vi "HFRR ADV v038.vi"() -> ()   [LabVIEW 2025] (continued)
            n2155 = Bundle "Bundle"(w2346, w2342) -> (w2348:cluster{dbl[], dbl[]})  [unwired: 1 in]
            n2156 = Bundle "Bundle"(w2311, w2310) -> (w2318:cluster{dbl[], dbl[]})  [unwired: 1 in]
            n2157 = Bundle "Bundle"(w2344, w2340) -> (w2350:cluster{dbl[], dbl[]})  [unwired: 1 in]
            n2158 = Bundle "Bundle"(w2311, w2344) -> (w2454:cluster{dbl[], dbl[]})  [unwired: 1 in]
            n2159 = Bundle "Bundle"(w2311, w2340) -> (w2378:cluster{dbl[], dbl[]})  [unwired: 1 in]
            n2160 = Bundle "Bundle"(w2311, w2399) -> (w2464:cluster{dbl[], dbl[]})  [unwired: 1 in]
            n2161 = Bundle "Bundle"(w2311, w2394) -> (w2402:cluster{dbl[], dbl[]})  [unwired: 1 in]
            n2162 = Bundle "Bundle"(w2311, w2425) -> (w2449:cluster{dbl[], dbl[]})  [unwired: 1 in]
            n2163 = Bundle "Bundle"(w2345, w2341) -> (w2349:cluster{dbl[], dbl[]})  [unwired: 1 in]
            n2164 = Bundle "Bundle"(w2313, w2312) -> (w2319:cluster{dbl[], dbl[]})  [unwired: 1 in]
            n2165 = Bundle "Bundle"(w2313, w2345) -> (w2456:cluster{dbl[], dbl[]})  [unwired: 1 in]
            n2166 = Bundle "Bundle"(w2313, w2341) -> (w2379:cluster{dbl[], dbl[]})  [unwired: 1 in]
            n2167 = Bundle "Bundle"(w2313, w2395) -> (w2403:cluster{dbl[], dbl[]})  [unwired: 1 in]
            n2168 = Bundle "Bundle"(w2313, w2397) -> (w2465:cluster{dbl[], dbl[]})  [unwired: 1 in]
            n2169 = Bundle "Bundle"(w2313, w2434) -> (w2447:cluster{dbl[], dbl[]})  [unwired: 1 in]
            n2170 = Bundle "Bundle"(w2343, w2339) -> (w2351:cluster{dbl[], dbl[]})  [unwired: 1 in]
            n2171 = Bundle "Bundle"(w2309, w2308) -> (w2317:cluster{dbl[], dbl[]})  [unwired: 1 in]
            n2172 = Bundle "Bundle"(w2309, w2343) -> (w2455:cluster{dbl[], dbl[]})  [unwired: 1 in]
            n2173 = Bundle "Bundle"(w2309, w2339) -> (w2377:cluster{dbl[], dbl[]})  [unwired: 1 in]
            n2174 = Bundle "Bundle"(w2309, w2393) -> (w2401:cluster{dbl[], dbl[]})  [unwired: 1 in]
            n2175 = Bundle "Bundle"(w2309, w2398) -> (w2463:cluster{dbl[], dbl[]})  [unwired: 1 in]
            n2176 = Bundle "Bundle"(w2309, w2416) -> (w2448:cluster{dbl[], dbl[]})  [unwired: 1 in]
            n2177 = call-poly <vilib>:"Mean.vi"("X"=w2396) -> ("mean"=→"CP1":dbl)  [unwired: 1 out]
            n2178 = call-poly <vilib>:"Mean.vi"("X"=w2337) -> ("mean"=→"КОФ2 3":dbl)  [unwired: 1 out]
            n2179 = call-poly <vilib>:"Mean.vi"("X"=w2395) -> ("mean"=→"CP2":dbl)  [unwired: 1 out]
            n2180 = call-poly <vilib>:"Mean.vi"("X"=w2397) -> ("mean"=→"КОФ2":dbl)  [unwired: 1 out]
            n2181 = call-poly <vilib>:"Mean.vi"("X"=w2335) -> ("mean"=→"КОФ2 5":dbl)  [unwired: 1 out]
            n2182 = call-poly <vilib>:"Mean.vi"("X"=w2393) -> ("mean"=→"CP4":dbl)  [unwired: 1 out]
            n2183 = call-poly <vilib>:"Mean.vi"("X"=w2398) -> ("mean"=→"КОФ4":dbl)  [unwired: 1 out]
            n2184 = Bundle "Bundle"(w2315, w2342) -> (w2306:cluster{dbl[], dbl[]})  [unwired: 1 in]
            n2185 = Bundle "Bundle"(w2315, w2396) -> (w2329:cluster{dbl[], dbl[]})  [unwired: 1 in]
            n2186 = Build Array "Build Array"(w2306, w2329) -> (w2332:cluster{dbl[], dbl[]}[])
            "XY Graph 17" <- w2332
            n2187 = Build Array "Build Array"(w2320, w2319, w2318, w2317) -> (→"Frequency ( Hz )":cluster{dbl[], dbl[]}[])
            n2188 = Build Array "Build Array"(w2348, w2349, w2350, w2351) -> (→"Air Temp ( °C ) vs Humidity ( % RH )":cluster{dbl[], dbl[]}[])
            n2189 = Build Array "Build Array"(w2333, w2456, w2454, w2455) -> (→"Air Temperature  ( °C )":cluster{dbl[], dbl[]}[])
            n2190 = Build Array "Build Array"(w2306, w2379, w2378, w2377) -> (→"Humidity ( %RH )":cluster{dbl[], dbl[]}[])
            n2191 = Build Array "Build Array"(w2334, w2465, w2464, w2463) -> (→"Coefficient Of Friction":cluster{dbl[], dbl[]}[])
            n2192 = Build Array "Build Array"(w2329, w2403, w2402, w2401) -> (→"Sample Temperature ( °C )":cluster{dbl[], dbl[]}[])
            n2193 = Build Array "Build Array"(w2307, w2447, w2449, w2448) -> (→"XY Graph 13":cluster{dbl[], dbl[]}[])
            n2194 = Bundle "Bundle"(w2315, w2338) -> (w2360:cluster{dbl[], dbl[]})  [unwired: 1 in]
            n2195 = Bundle "Bundle"(w2311, w2336) -> (w2358:cluster{dbl[], dbl[]})  [unwired: 1 in]
            n2196 = Bundle "Bundle"(w2313, w2337) -> (w2359:cluster{dbl[], dbl[]})  [unwired: 1 in]
            n2197 = Bundle "Bundle"(w2309, w2335) -> (w2357:cluster{dbl[], dbl[]})  [unwired: 1 in]
            n2198 = Build Array "Build Array"(w2360, w2359, w2358, w2357) -> (→"Stroke ( mm )":cluster{dbl[], dbl[]}[])
            n2199 = local write "XY Graph 16"(w2332) -> ()
          }
          frame #2 {
          }
          frame #3 {
            n2200 = local write "Numeric 8"(0 ("Numeric 8")) -> ()
            n2201 = local write "Numeric 11"(0 ("Numeric 11")) -> ()
            n2202 = local write "Numeric 12"(0 ("Numeric 12")) -> ()
            n2203 = local write "Numeric 13"(0 ("Numeric 13")) -> ()
            n2204 = property on="OPEN" class="Bool (strict)"("Visible"=TRUE) -> ()  [unwired: 2 in, 2 out]
            n2205 = local read "String Control 2"() -> (w2632:string)
            n2206 = local read "String Control 4"() -> (w2631:string)
            n2207 = local read "String Control 6"() -> (w2630:string)
            n2208 = local read "String Control 8"() -> (w2629:string)
            n2209 = Match Pattern(string=w2632, regular expression="Samples / cycle :- ") -> (after substring=w2646:string)  [unwired: 1 in, 3 out]
            n2210 = Match Pattern(string=w2632, regular expression="Frequency :- ") -> (after substring=w2665:string)  [unwired: 1 in, 3 out]
            n2211 = Match Pattern(string=w2631, regular expression="Samples / cycle :- ") -> (after substring=w2642:string)  [unwired: 1 in, 3 out]
            n2212 = Match Pattern(string=w2631, regular expression="Frequency :- ") -> (after substring=w2660:string)  [unwired: 1 in, 3 out]
            n2213 = Match Pattern(string=w2630, regular expression="Samples / cycle :- ") -> (after substring=w2638:string)  [unwired: 1 in, 3 out]
            n2214 = Match Pattern(string=w2630, regular expression="Frequency :- ") -> (after substring=w2655:string)  [unwired: 1 in, 3 out]
            n2215 = Match Pattern(string=w2629, regular expression="Samples / cycle :- ") -> (after substring=w2634:string)  [unwired: 1 in, 3 out]
            n2216 = Match Pattern(string=w2629, regular expression="Frequency :- ") -> (after substring=w2650:string)  [unwired: 1 in, 3 out]
            n2217 = String Subset(string=w2646, length (rest)=6 ("length (rest)")) -> (substring=w2648:string)  [unwired: 1 in]
            n2218 = String Subset(string=w2665, length (rest)=9 ("length (rest)")) -> (substring=w2667:string)  [unwired: 1 in]
            n2219 = String Subset(string=w2642, length (rest)=6 ("length (rest)")) -> (substring=w2644:string)  [unwired: 1 in]
            n2220 = String Subset(string=w2660, length (rest)=9 ("length (rest)")) -> (substring=w2662:string)  [unwired: 1 in]
            n2221 = String Subset(string=w2638, length (rest)=6 ("length (rest)")) -> (substring=w2640:string)  [unwired: 1 in]
            n2222 = String Subset(string=w2655, length (rest)=9 ("length (rest)")) -> (substring=w2657:string)  [unwired: 1 in]
            n2223 = String Subset(string=w2634, length (rest)=6 ("length (rest)")) -> (substring=w2636:string)  [unwired: 1 in]
            n2224 = String Subset(string=w2650, length (rest)=9 ("length (rest)")) -> (substring=w2652:string)  [unwired: 1 in]
            n2225 = Fract/Exp String To Number(string=w2648) -> (number=w2628:dbl)  [unwired: 3 in, 1 out]
            n2226 = Fract/Exp String To Number(string=w2667) -> (number=w2668:dbl)  [unwired: 3 in, 1 out]
            n2227 = Fract/Exp String To Number(string=w2644) -> (number=w2627:dbl)  [unwired: 3 in, 1 out]
            n2228 = Fract/Exp String To Number(string=w2662) -> (number=w2663:dbl)  [unwired: 3 in, 1 out]
            n2229 = Fract/Exp String To Number(string=w2640) -> (number=w2626:dbl)  [unwired: 3 in, 1 out]
            n2230 = Fract/Exp String To Number(string=w2657) -> (number=w2658:dbl)  [unwired: 3 in, 1 out]
            n2231 = Fract/Exp String To Number(string=w2636) -> (number=w2625:dbl)  [unwired: 3 in, 1 out]
            n2232 = Fract/Exp String To Number(string=w2652) -> (number=w2653:dbl)  [unwired: 3 in, 1 out]
            n2233 = local write "sample1"(w2628) -> ()
            n2234 = local write "freq1"(w2668) -> ()
            n2235 = local write "sample2"(w2627) -> ()
            n2236 = local write "freq2"(w2663) -> ()
            n2237 = local write "sample3"(w2626) -> ()
            n2238 = local write "freq3"(w2658) -> ()
            n2239 = local write "sample4"(w2625) -> ()
            n2240 = local write "freq 4"(w2653) -> ()
          }
        }
      }
    }
    n2241 = case shown="True" w2226 {
      selector: w2226 -> [_ w2245]
      frame False {
      }
      frame True {
        n2242 = Not(x=w2245) -> (.not. x?=w2241:bool)
        n2243 = local write "service 3"(w2241) -> ()
        n2244 = local write "OPEN 6"(w2241) -> ()
        n2245 = call <vilib>:"System Exec.vi"("wait until completion? (T)"=TRUE, "command line"="C:\\LAB-IQ\\Scar View.exe") -> ("error out"=→"error out 5":errorcluster)  [unwired: 6 in, 3 out]
      }
    }
    n2246 = case shown="\"Acquire\", Default" w2235 {
      frame "Acquire", Default {
        # "Elapsed time\ncof\nstroke\nAir temp\nTemp\nHumidity"
        n2247 = disable-structure shown="Disabled" {
          frame Disabled {
            n2248 = local read "Flag"() -> (w2944:dbl)
            n2249 = local read "RUN"() -> (w2941:bool)
            n2250 = Not(x=w2941) -> (.not. x?=w2940:bool)
            n2251 = Equal?(x=w2944, y=10.0) -> (x = y?=w2942:bool)
            n2252 = And(x=w2942, y=w2940) -> (x .and. y?=w2939:bool)
            n2253 = case shown="True" w2939 {
              frame False {
              }
              frame True {
                w2945 = FALSE ("Heater Button")
                n2254 = local write "Humidity"(w2945) -> ()
                n2255 = local write "Heater Button"(w2945) -> ()
              }
            }
          }
          frame Enabled {
          }
        }
        n2256 = disable-structure shown="Disabled" {
          frame Disabled {
            n2257 = case shown="True" {
              selector: _ -> [_ _]
              frame False {
              }
              frame True {
                w2990 = TRUE ("Heater")
                n2258 = local write "Humidity"(w2990) -> ()
                n2259 = local write "Heater Button"(w2990) -> ()
                n2260 = local read "TEST STANDARD"() -> (w2993:T3)
                n2261 = local read "TEST STANDARD"() -> (w2988:T3)
                n2262 = Equal?(x=w2993, y=enum16{"ASTM D6079", "ISO 12156", "Custom"}."ISO 12156" ("Test Standard")) -> (x = y?=w2991:bool)
                n2263 = Equal?(x=w2988, y=enum16{"ASTM D6079", "ISO 12156", "Custom"}."ASTM D6079" ("Test Standard")) -> (x = y?=w2987:bool)
                n2264 = case shown="True" w2991 {
                  frame False {
                  }
                  frame True {
                    n2265 = local write "airtempflg"(FALSE ("airtempflg")) -> ()
                    n2266 = local write item#-1(TRUE ("Heater")) -> ()
                  }
                }
                n2267 = case shown="True" w2987 {
                  frame False {
                  }
                  frame True {
                    n2268 = local write "airtempflg"(TRUE ("airtempflg")) -> ()
                    n2269 = local write item#-1(FALSE ("Heater")) -> ()
                  }
                }
              }
            }
          }
          frame Enabled {
          }
        }
        n2270 = stacked-sequence {
          frame #0 {
            n2271 = case shown="True" "RST FF" {
              frame False {
              }
              frame True {
                w3007 = 0.0 ("X Scale.Range:Maximum")
                n2272 = property on="Frictional Force ( N )" class="WFChart (strict)"("XScale.Maximum"=600.0 ("X Scale.Range:Maximum"), "XScale.Minimum"=w3007, "YScale.Maximum"=10.0 ("Y Scale.Range:Maximum"), "YScale.Minimum"=w3007) -> ()  [unwired: 2 in, 2 out]
              }
            }
          }
          frame #1 {
            n2273 = case shown="True" "RST TEMP" {
              frame False {
              }
              frame True {
                n2274 = property on="Temperature ( Deg C )" class="WFChart (strict)"("XScale.Minimum"=0.0 ("X Scale.Range:Minimum"), "XScale.Maximum"=600.0 ("X Scale.Range:Maximum"), "YScale.Minimum"=0.0 ("Y Scale.Range:Minimum"), "YScale.Maximum"=100.0 ("Y Scale.Range:Maximum")) -> ()  [unwired: 2 in, 2 out]
              }
            }
          }
          frame #2 {
            n2275 = case shown="True" "RSTCOF" {
              frame False {
              }
              frame True {
                n2276 = property on="Coefficient of Friction" class="WFChart (strict)"("XScale.Minimum"=0.0 ("X Scale.Range:Minimum"), "XScale.Maximum"=600.0 ("X Scale.Range:Maximum"), "YScale.Maximum"=1.0 ("X Scale.Range:Minimum"), "YScale.Minimum"=0.0 ("X Scale.Range:Minimum")) -> ()  [unwired: 2 in, 2 out]
              }
            }
          }
          frame #3 {
            n2277 = case shown="True" "RSTCOF 2" {
              frame False {
              }
              frame True {
                (unwired) 100.0 ("Y Scale.Range:Maximum")
                (unwired) 0.0 ("Y Scale.Range:Minimum")
                (unwired) 600.0 ("X Scale.Range:Maximum")
                (unwired) 0.0 ("X Scale.Range:Minimum")
              }
            }
          }
          frame #4 {
            n2278 = case shown="True" "RSTCOF 3" {
              frame False {
              }
              frame True {
                n2279 = property on="Electrical Contact Resistance ( % )" class="WFChart (strict)"("XScale.Minimum"=0.0 ("X Scale.Range:Minimum"), "XScale.Maximum"=600.0 ("X Scale.Range:Maximum"), "YScale.Minimum"=0.0 ("Y Scale.Range:Minimum"), "YScale.Maximum"=100.0 ("Y Scale.Range:Maximum")) -> ()  [unwired: 2 in, 2 out]
              }
            }
          }
        }
        n2280 = local read "RUN"() -> (w2934:bool)
        n2281 = case shown="False" w2934 {
          frame False {
          }
          frame True {
          }
        }
        n2282 = local read "RUN"() -> (w2938:bool)
        n2283 = case shown="False" w2938 {
          tunnel: [FALSE ("TEST RUNNING") TRUE ("TEST RUNNING")] -> w2937
          frame False {
            w3026 = 0.0 ("Flag")
            n2284 = local write "Elapsed time"(0.0 ("elapsedtime")) -> ()
            n2285 = local write "Time Remaining"(w3026) -> ()
            n2286 = local write "Flag"(w3026) -> ()
            n2287 = local write "Remaining Time"(w3026) -> ()
          }
          frame True {
            n2288 = local write "Flag"(10.0 ("Flag")) -> ()
          }
        }
        n2289 = local read "AIR TEMP"() -> (w2932:dbl)
        n2290 = Greater Or Equal?(x=w2932, y=15.0) -> (x >= y?=w2933:bool)
        "powstat" <- w2933
        n2291 = case shown="True" "Save & Continue" {
          frame False {
          }
          frame True {
            n2292 = local read "USER ID"() -> (w3330:string)
            n2293 = local read "FILE"() -> (w3338:string)
            n2294 = String Length(string=w3338) -> (length=w3336:i32)
            n2295 = String Length(string=w3330) -> (length=w3333:i32)
            n2296 = Greater?(x=w3336, y=0) -> (0:w3335:bool)
            n2297 = Greater?(x=w3333, y=0) -> (0:w3332:bool)
            n2298 = And(x=w3335, y=w3332) -> (x .and. y?=w3331:bool)
            n2299 = case shown="True" w3331 {
              frame False {
                n2300 = stacked-sequence {
                  frame #0 {
                    n2301 = One Button Dialog(message="Please Enter a File Name and Operator ID to save data !", button name ("OK")="Ok") -> ()  [unwired: 1 out]
                  }
                  frame #1 {
                    n2302 = local write "Save & Continue"(FALSE ("OK Button")) -> ()
                  }
                }
                n2303 = local write "Save & Continue"(FALSE ("OK Button")) -> ()
              }
              frame True {
                n2304 = stacked-sequence {
                  frame #0 {
                    n2305 = local read "FILE"() -> (w3344:string)
                    n2306 = call "file check.vi"("file name in"=w3344) -> ("file name out"=w3343:string)  [unwired: 9 in, 1 out]
                    n2307 = call <vilib>:"Application Directory.vi"() -> ("Application Directory"=w3354:path)
                    n2308 = Build Path(base path=w3354, name or relative path="data") -> (appended path=w3353:path)
                    n2309 = call <vilib>:"Trim Whitespace.vi"("string"=w3343) -> ("trimmed string"=w3351:string)  [unwired: 1 in]
                    n2310 = call <vilib>:"Trim Whitespace.vi"("string"=w3343) -> ("trimmed string"=w3352:string)  [unwired: 1 in]
                    n2311 = List Folder(path=w3353) -> (folder names=w3349:string[])  [unwired: 3 in, 3 out]
                    n2312 = Match Pattern(string=w3351, regular expression="_(") -> (before substring=w3348:string)  [unwired: 1 in, 3 out]
                    n2313 = for {
                      tunnel: w3349 -> [w3363] mode=indexing
                      tunnel: w3348 -> [w3361]
                      shift-right: [w3359] -> w3346
                      shift-left: bool[] [] -> [w3360]
                      n2314 = Match Pattern(string=w3363, regular expression="_(") -> (before substring=w3362:string)  [unwired: 1 in, 3 out]
                      n2315 = Equal?(x=w3362, y=w3361) -> (x = y?=w3358:bool)
                      n2316 = case shown="True" w3358 {
                        tunnel: w3358 -> [_ w3366]
                        tunnel: w3360 -> [w3365 w3368]
                        tunnel: [w3365 w3367] -> w3359
                        frame False {
                        }
                        frame True {
                          n2317 = Insert Into Array(array=w3368, new element=w3366) -> (w3367:bool[])  [unwired: 1 in]
                        }
                      }
                    }
                    n2318 = Equal?(x=w3349, y=w3348) -> (x = y?=w3357:bool[])
                    n2319 = Or Array Elements(Boolean array=w3357) -> (logical OR=w3356:bool)
                    n2320 = Array Size(array=w3346) -> (size(s)=w3345:i32)
                    n2321 = case shown="True" w3356 {
                      tunnel: w3352 -> [_ w3376]
                      tunnel: w3345 -> [_ w3369]
                      frame False {
                      }
                      frame True {
                        n2322 = Number To Decimal String(number=w3369) -> (decimal integer string=w3372:string)  [unwired: 1 in]
                        n2323 = Search/Split String(string=w3376, search string/char (-)="_(" ("regular expression")) -> (substring before match=w3374:string)  [unwired: 1 in, 2 out]
                        n2324 = Concatenate Strings(w3374, "_(" ("regular expression"), w3372, ")" ("regular expression")) -> (w3370:string)
                        n2325 = local write "FILE"(w3370) -> ()
                      }
                    }
                  }
                  frame #1 {
                    w3379 = 0.0
                    w3392 = cluster{"y":dbl, dbl, "y":dbl}[] [] ("History Data")
                    w3393 = FALSE ("Heater Button")
                    (unwired) ")!" ("string")
                    (unwired) ")" ("string")
                    w3391 = dbl[] [] ("History Data")
                    w3397 = "\r"
                    # "C:\\WinDucom\\Data\\"
                    # "C:\\LAB-IQ-NXT\\data"
                    n2326 = local write "Humidity ( %RH )"(w3379) -> ()
                    n2327 = local write "Frequency ( Hz )"(w3379) -> ()
                    n2328 = local write "Stroke 3"(w3379) -> ()
                    n2329 = local write "speedop"(0.0 ("PIDclk 2")) -> ()
                    n2330 = local write "Set Temp 2"(65.0 ("Set Temp 2")) -> ()
                    n2331 = local write "AIR TEMP"(w3379) -> ()
                    n2332 = local write "clk"(0.0 ("clk")) -> ()
                    n2333 = local write "Stroke 4"(w3379) -> ()
                    n2334 = local write "COF 2"(w3379) -> ()
                    n2335 = local write "TEMP"(w3379) -> ()
                    n2336 = local write "ecr 3"(w3379) -> ()
                    n2337 = local write "FF 3"(w3379) -> ()
                    n2338 = local write "FF 2"(w3379) -> ()
                    n2339 = property on="Coefficient of Friction" class="WFChart (strict)"("History Data"=w3391) -> ()  [unwired: 2 in, 2 out]
                    n2340 = property on="Coefficient of Friction" class="WFChart (strict)"("History Data"=w3391) -> ()  [unwired: 2 in, 2 out]
                    n2341 = property on="Frictional Force ( N )" class="WFChart (strict)"("History Data"=w3391) -> ()  [unwired: 2 in, 2 out]
                    n2342 = property on="Electrical Contact Resistance ( % )" class="WFChart (strict)"("History Data"=w3391) -> ()  [unwired: 2 in, 2 out]
                    n2343 = property on="Electrical Contact Resistance ( % )" class="WFChart (strict)"("History Data"=w3391) -> ()  [unwired: 2 in, 2 out]
                    n2344 = property on="Temperature ( Deg C )" class="WFChart (strict)"("History Data"=w3391) -> ()  [unwired: 2 in, 2 out]
                    n2345 = property on="Frictional Force ( N )" class="WFChart (strict)"("History Data"=w3391) -> ()  [unwired: 2 in, 2 out]
                    n2346 = property on="Coefficient of Friction" class="WFChart (strict)"("History Data"=w3391) -> ()  [unwired: 2 in, 2 out]
                    n2347 = property on="Frictional Force ( N )" class="WFChart (strict)"("History Data"=w3391) -> ()  [unwired: 2 in, 2 out]
                    n2348 = property on="Electrical Contact Resistance ( % )" class="WFChart (strict)"("History Data"=w3391) -> ()  [unwired: 2 in, 2 out]
                    n2349 = property on="Temperature ( Deg C )" class="WFChart (strict)"("History Data"=w3391) -> ()  [unwired: 2 in, 2 out]
                    n2350 = property on="Stroke ( mm )" class="WFChart (strict)"("History Data"=w3392) -> ()  [unwired: 2 in, 2 out]
                    n2351 = property on="Stroke ( mm )" class="WFChart (strict)"("History Data"=w3392) -> ()  [unwired: 2 in, 2 out]
                    n2352 = local write "Humidity"(w3393) -> ()
                    n2353 = local write "Heater Button"(w3393) -> ()
                    n2354 = local read "FILE"() -> (w3387:string)
                    n2355 = disable-structure shown="Enabled" {
                      disable-tunnel: [w3431 _] -> w3378
                      frame Enabled {
                        n2356 = local read "NORMAL LOAD"() -> (w3431:dbl)
                      }
                      frame Disabled {
                      }
                    }
                    n2357 = call "file check.vi"("file name in"=w3387) -> ("error out"=w3390:errorcluster, "file name out"=w3384:string)  [unwired: 9 in]
                    n2358 = call "FILE PATH CREATION.vi"("error in"=w3390, "FILE NAME :"=w3384) -> ("FILE OUT"=w3383:path)  [unwired: 8 in, 1 out]
                    n2359 = Concatenate Strings(w3384, ".dgf" ("Substring")) -> (w3389:string)
                    n2360 = Concatenate Strings(w3384, ".duf" ("Substring")) -> (w3385:string)
                    n2361 = Multiply(x=w3378, y=1.0) -> (x*y=w3410:dbl)
                    n2362 = Build Path(base path=w3383, name or relative path=w3389) -> (appended path=w3382:path)
                    n2363 = Build Path(base path=w3383, name or relative path=w3385) -> (appended path=w3381:path)
                    n2364 = Number To Fractional String(number=w3410, width (-)=i16 5, precision (6)=i16 2) -> (F-format string=w3418:string)  [unwired: 1 in]
                    n2365 = local read "tested by"() -> (w3377:string)
                    n2366 = local read "Fuel Discription :"() -> (w3406:string)
                    n2367 = local read "Batch Ref Num :"() -> (w3395:string)
                    n2368 = Get Date/Time String(date format (0)=enum16{"short", "long", "abbreviated"}."short") -> (date string=w3429:string, time string=w3426:string)  [unwired: 2 in]
                    n2369 = local read "Remarks :"() -> (w3405:string)
                    n2370 = Concatenate Strings("Load :- " ("Substring"), w3418, " grams ," ("Substring")) -> (w3417:string)
                    n2371 = local read "String 41"() -> (w3398:string)
                    n2372 = Concatenate Strings(w3406) -> (w3407:string)
                    n2373 = Concatenate Strings(w3395) -> (w3394:string)
                    n2374 = Concatenate Strings(w3377) -> (w3401:string)
                    n2375 = Concatenate Strings("(" ("Substring"), w3429, ")" ("Substring"), w3426) -> (w3400:string)
                    "concatenated string" <- w3400
                    n2376 = Concatenate Strings(w3405, "," ("string")) -> (w3404:string)
                    n2377 = Concatenate Strings("  TIME;      COF;       STROKE;     AIR TEMP;  TEMP;  HUMIDITY;  ECR; PID-OUT; FREQUENCY" ("Substring"), "\r") -> (w3413:string)
                    n2378 = Concatenate Strings(w3398, w3397, "Fuel Discription :-" ("Substring"), w3407, w3397, w3417, w3397, "Batch Ref Num :-" ("Substring"), w3394, w3397, " Remarks :- " ("Substring"), w3404, w3397, " Date :- " ("Substring"), w3400, w3397, "Tested By :-" ("Substring"), w3401) -> (w3411:string)
                    "REMARKS" <- w3411
                    n2379 = call <vilib>:"Write Characters To File.vi"("append to file? (new file:F)"=FALSE, "character string"=w3413, "file path (dialog if empty)"=w3382) -> ()  [unwired: 2 in, 1 out]
                    n2380 = call <vilib>:"Write Characters To File.vi"("append to file? (new file:F)"=FALSE, "character string"=w3411, "file path (dialog if empty)"=w3381) -> ()  [unwired: 2 in, 1 out]
                  }
                  frame #2 {
                    n2381 = local write "Cycles elapsed"(0 ("Cycles elapsed")) -> ()
                    n2382 = local write "cyclecount"(0 ("cyclecount")) -> ()
                    n2383 = local write "Save & Continue"(FALSE ("OK")) -> ()
                    n2384 = local write "autostrtflg"(TRUE ("autostrtflg")) -> ()
                    n2385 = local write "Save"(FALSE ("Save")) -> ()
                    n2386 = Get Date/Time In Seconds() -> (seconds since 1Jan1904=w3436:timestamp)
                    n2387 = To Double Precision Float(number=w3436) -> (double precision float=w3435:dbl)
                    n2388 = local write "acq timer"(w3435) -> ()
                    n2389 = One Button Dialog(message="Please ensure sample is mounted properly and machine is ready in all aspects for testing !", button name ("OK")="Ok") -> ()  [unwired: 1 out]
                  }
                  frame #3 {
                    n2390 = stacked-sequence {
                      frame #0 {
                        n2391 = local write "Main Dashboard Buttons"(T1."Dashboard" ("Main Dashboard Buttons")) -> ()
                        n2392 = local write "Main Tab"(T2."Acquire" ("Main Tab")) -> ()
                      }
                      frame #1 {
                        n2393 = local write "EVENT LOG"("" ("EVENT LOG")) -> ()
                      }
                      frame #2 {
                        n2394 = Wait (ms)(milliseconds to wait=u32 50) -> ()  [unwired: 1 out]
                      }
                      frame #3 {
                        n2395 = disable-structure shown="Disabled" {
                          frame Disabled {
                            n2396 = local read "EVENT LOG"() -> (w3448:string)
                            n2397 = call "Event Log.vi"("Content"="Test Details", "EVENT LOG"=w3448) -> ("EVENT LOG"=w3447:string)  [unwired: 8 in, 1 out]
                            n2398 = local write "EVENT LOG"(w3447) -> ()
                          }
                          frame Enabled {
                          }
                        }
                      }
                      frame #4 {
                        n2399 = Wait (ms)(milliseconds to wait=u32 50) -> ()  [unwired: 1 out]
                      }
                      frame #5 {
                        n2400 = local read "FILE"() -> (w3450:string)
                        n2401 = Concatenate Strings("File Name :" ("Content"), w3450) -> (w3451:string)
                        n2402 = local read "EVENT LOG"() -> (w3454:string)
                        n2403 = call "Event Log.vi"("Content"=w3451, "EVENT LOG"=w3454) -> ("EVENT LOG"=w3453:string)  [unwired: 8 in, 1 out]
                        n2404 = local write "EVENT LOG"(w3453) -> ()
                      }
                      frame #6 {
                        n2405 = Wait (ms)(milliseconds to wait=u32 50) -> ()  [unwired: 1 out]
                      }
                      frame #7 {
                        n2406 = local read "Batch Ref Num :"() -> (w3456:string)
                        n2407 = Concatenate Strings("Batch Ref No :" ("Content"), w3456) -> (w3457:string)
                        n2408 = local read "EVENT LOG"() -> (w3460:string)
                        n2409 = call "Event Log.vi"("Content"=w3457, "EVENT LOG"=w3460) -> ("EVENT LOG"=w3459:string)  [unwired: 8 in, 1 out]
                        n2410 = local write "EVENT LOG"(w3459) -> ()
                      }
                      frame #8 {
                        n2411 = Wait (ms)(milliseconds to wait=u32 50) -> ()  [unwired: 1 out]
                      }
                      frame #9 {
                        n2412 = local read "tested by"() -> (w3462:string)
                        n2413 = Concatenate Strings("Tested By :" ("Content"), w3462) -> (w3463:string)
                        n2414 = local read "EVENT LOG"() -> (w3466:string)
                        n2415 = call "Event Log.vi"("Content"=w3463, "EVENT LOG"=w3466) -> ("EVENT LOG"=w3465:string)  [unwired: 8 in, 1 out]
                        n2416 = local write "EVENT LOG"(w3465) -> ()
                      }
                      frame #10 {
                        n2417 = Wait (ms)(milliseconds to wait=u32 50) -> ()  [unwired: 1 out]
                      }
                      frame #11 {
                        n2418 = local read "TEST STANDARD"() -> (w3469:T3)
                        n2419 = case shown="\"ASTM D6079\", Default" w3469 {
                          tunnel: ["ASTM D6079" "ISO 12156" "CEC F-096-A-06" "Custom"] -> w3468
                          frame "ASTM D6079", Default {
                          }
                          frame "ISO 12156" {
                          }
                          frame "CEC F-096-A-06" {
                          }
                          frame "Custom" {
                          }
                        }
                        n2420 = Concatenate Strings("Test Standard :" ("Content"), w3468) -> (w3470:string)
                        n2421 = local read "EVENT LOG"() -> (w3473:string)
                        n2422 = call "Event Log.vi"("Content"=w3470, "EVENT LOG"=w3473) -> ("EVENT LOG"=w3472:string)  [unwired: 8 in, 1 out]
                        n2423 = local write "EVENT LOG"(w3472) -> ()
                      }
                      frame #12 {
                        n2424 = Wait (ms)(milliseconds to wait=u32 50) -> ()  [unwired: 1 out]
                      }
                      frame #13 {
                        n2425 = local read "Fuel Discription :"() -> (w3479:string)
                        n2426 = Concatenate Strings("Fuel Description :" ("Content"), w3479) -> (w3480:string)
                        n2427 = local read "EVENT LOG"() -> (w3483:string)
                        n2428 = call "Event Log.vi"("Content"=w3480, "EVENT LOG"=w3483) -> ("EVENT LOG"=w3482:string)  [unwired: 8 in, 1 out]
                        n2429 = local write "EVENT LOG"(w3482) -> ()
                      }
                      frame #14 {
                        n2430 = Wait (ms)(milliseconds to wait=u32 50) -> ()  [unwired: 1 out]
                      }
                      frame #15 {
                        n2431 = local read "Remarks :"() -> (w3485:string)
                        n2432 = Concatenate Strings("Remarks :" ("Content"), w3485) -> (w3486:string)
                        n2433 = local read "EVENT LOG"() -> (w3489:string)
                        n2434 = call "Event Log.vi"("Content"=w3486, "EVENT LOG"=w3489) -> ("EVENT LOG"=w3488:string)  [unwired: 8 in, 1 out]
                        n2435 = local write "EVENT LOG"(w3488) -> ()
                      }
                      frame #16 {
                        n2436 = Wait (ms)(milliseconds to wait=u32 50) -> ()  [unwired: 1 out]
                      }
                      frame #17 {
                        n2437 = local read "USER ID"() -> (w3491:string)
                        n2438 = Concatenate Strings("Operator ID :" ("Content"), w3491) -> (w3493:string)
                        n2439 = local read "EVENT LOG"() -> (w3495:string)
                        n2440 = call "Event Log.vi"("Content"=w3493, "EVENT LOG"=w3495) -> ("EVENT LOG"=w3494:string)  [unwired: 8 in, 1 out]
                        n2441 = local write "EVENT LOG"(w3494) -> ()
                      }
                      frame #18 {
                        n2442 = Wait (ms)(milliseconds to wait=u32 50) -> ()  [unwired: 1 out]
                      }
                      frame #19 {
                        n2443 = disable-structure shown="Disabled" {
                          frame Disabled {
                            n2444 = local read "EVENT LOG"() -> (w3499:string)
                            n2445 = call "Event Log.vi"("Content"="Test Parameter", "EVENT LOG"=w3499) -> ("EVENT LOG"=w3498:string)  [unwired: 8 in, 1 out]
                            n2446 = local write "EVENT LOG"(w3498) -> ()
                          }
                          frame Enabled {
                          }
                        }
                      }
                      frame #20 {
                        n2447 = Wait (ms)(milliseconds to wait=u32 50) -> ()  [unwired: 1 out]
                      }
                      frame #21 {
                        n2448 = local read "Set Hz"() -> (w3503:dbl)
                        n2449 = Number To Fractional String(number=w3503, precision (6)=i16 2) -> (F-format string=w3502:string)  [unwired: 2 in]
                        n2450 = Concatenate Strings("Set Frequency [Hz] :" ("Content"), w3502) -> (w3505:string)
                        n2451 = local read "EVENT LOG"() -> (w3507:string)
                        n2452 = call "Event Log.vi"("Content"=w3505, "EVENT LOG"=w3507) -> ("EVENT LOG"=w3506:string)  [unwired: 8 in, 1 out]
                        n2453 = local write "EVENT LOG"(w3506) -> ()
                      }
                      frame #22 {
                        n2454 = Wait (ms)(milliseconds to wait=u32 50) -> ()  [unwired: 1 out]
                      }
                      frame #23 {
                        n2455 = local read "NORMAL LOAD"() -> (w3510:dbl)
                        n2456 = Number To Fractional String(number=w3510, precision (6)=i16 2) -> (F-format string=w3511:string)  [unwired: 2 in]
                        n2457 = Concatenate Strings("Applied Load [grams] :" ("Content"), w3511) -> (w3513:string)
                        n2458 = local read "EVENT LOG"() -> (w3515:string)
                        n2459 = call "Event Log.vi"("Content"=w3513, "EVENT LOG"=w3515) -> ("EVENT LOG"=w3514:string)  [unwired: 8 in, 1 out]
                        n2460 = local write "EVENT LOG"(w3514) -> ()
                      }
                      frame #24 {
                        n2461 = Wait (ms)(milliseconds to wait=u32 50) -> ()  [unwired: 1 out]
                      }
                      frame #25 {
                        n2462 = local read "Set Strk"() -> (w3518:dbl)
                        n2463 = Number To Fractional String(number=w3518, precision (6)=i16 2) -> (F-format string=w3519:string)  [unwired: 2 in]
                        n2464 = Concatenate Strings("Set Stroke [mm] :" ("Content"), w3519) -> (w3521:string)
                        n2465 = local read "EVENT LOG"() -> (w3523:string)
                        n2466 = call "Event Log.vi"("Content"=w3521, "EVENT LOG"=w3523) -> ("EVENT LOG"=w3522:string)  [unwired: 8 in, 1 out]
                        n2467 = local write "EVENT LOG"(w3522) -> ()
                      }
                      frame #26 {
                        n2468 = Wait (ms)(milliseconds to wait=u32 50) -> ()  [unwired: 1 out]
                      }
                      frame #27 {
                        n2469 = local read "Set Temp"() -> (w3526:dbl)
                        n2470 = Number To Fractional String(number=w3526, precision (6)=i16 2) -> (F-format string=w3527:string)  [unwired: 2 in]
                        n2471 = Concatenate Strings("Set Temperature [deg C] :" ("Content"), w3527) -> (w3529:string)
                        n2472 = local read "EVENT LOG"() -> (w3531:string)
                        n2473 = call "Event Log.vi"("Content"=w3529, "EVENT LOG"=w3531) -> ("EVENT LOG"=w3530:string)  [unwired: 8 in, 1 out]
                        n2474 = local write "EVENT LOG"(w3530) -> ()
                      }
                      frame #28 {
                        n2475 = Wait (ms)(milliseconds to wait=u32 50) -> ()  [unwired: 1 out]
                      }
                      frame #29 {
                        n2476 = local read "Set Rh"() -> (w3534:dbl)
                        n2477 = Number To Fractional String(number=w3534, precision (6)=i16 2) -> (F-format string=w3535:string)  [unwired: 2 in]
                        n2478 = Concatenate Strings("Set Humidity [%RH] :" ("Content"), w3535) -> (w3537:string)
                        n2479 = local read "EVENT LOG"() -> (w3539:string)
                        n2480 = call "Event Log.vi"("Content"=w3537, "EVENT LOG"=w3539) -> ("EVENT LOG"=w3538:string)  [unwired: 8 in, 1 out]
                        n2481 = local write "EVENT LOG"(w3538) -> ()
                      }
                      frame #30 {
                        n2482 = Wait (ms)(milliseconds to wait=u32 50) -> ()  [unwired: 1 out]
                      }
                      frame #31 {
                        n2483 = local read "test time"() -> (w3542:dbl)
                        n2484 = Number To Fractional String(number=w3542, precision (6)=i16 1) -> (F-format string=w3543:string)  [unwired: 2 in]
                        n2485 = Concatenate Strings("Test Duration [mins] :" ("Content"), w3543) -> (w3545:string)
                        n2486 = local read "EVENT LOG"() -> (w3547:string)
                        n2487 = call "Event Log.vi"("Content"=w3545, "EVENT LOG"=w3547) -> ("EVENT LOG"=w3546:string)  [unwired: 8 in, 1 out]
                        n2488 = local write "EVENT LOG"(w3546) -> ()
                      }
                      frame #32 {
                        w3548 = dbl[] [] ("History Data")
                        w3549 = cluster{"y":dbl, dbl, "y":dbl}[] [] ("History Data")
                        w3550 = FALSE ("Visible")
                        n2489 = property on="Stroke ( mm )" class="WFChart (strict)"("History Data"=w3549) -> ()  [unwired: 2 in, 2 out]
                        n2490 = property on="Temperature ( Deg C )" class="WFChart (strict)"("History Data"=w3548) -> ()  [unwired: 2 in, 2 out]
                        n2491 = property on="Electrical Contact Resistance ( % )" class="WFChart (strict)"("History Data"=w3548) -> ()  [unwired: 2 in, 2 out]
                        n2492 = property on="Coefficient of Friction" class="WFChart (strict)"("History Data"=w3548) -> ()  [unwired: 2 in, 2 out]
                        n2493 = property on="Frictional Force ( N )" class="WFChart (strict)"("History Data"=w3548) -> ()  [unwired: 2 in, 2 out]
                        n2494 = property on="Coefficient of Friction" class="WFChart (strict)"("History Data"=w3548) -> ()  [unwired: 2 in, 2 out]
                        n2495 = property on="Frictional Force ( N )" class="WFChart (strict)"("History Data"=w3548) -> ()  [unwired: 2 in, 2 out]
                        n2496 = property on="Electrical Contact Resistance ( % )" class="WFChart (strict)"("History Data"=w3548) -> ()  [unwired: 2 in, 2 out]
                        n2497 = property on="Stroke ( mm )" class="WFChart (strict)"("History Data"=w3549) -> ()  [unwired: 2 in, 2 out]
                        n2498 = property on="Temperature ( Deg C )" class="WFChart (strict)"("History Data"=w3548) -> ()  [unwired: 2 in, 2 out]
                        n2499 = property on="Service Password Log" class="Str"("Visible"=w3550) -> ()  [unwired: 2 in, 2 out]
                        n2500 = property on="Password 3" class="Clust (strict)"("Visible"=w3550) -> ()  [unwired: 2 in, 2 out]
                      }
                    }
                    "TEST FILE NAM,E SAVED" <- TRUE ("TEST FILE NAM,E SAVED")
                  }
                }
              }
            }
          }
        }
        n2501 = local write "Test \nStatus"(w2937) -> ()
        n2502 = local write "Save"(w2937) -> ()
        n2503 = local read "Main Tab"() -> (w2931:T2)
        n2504 = case shown="True" w2934 {
          frame False {
            n2505 = local read "Rt 3"() -> (w2998:bool)
            n2506 = case shown="True" w2998 {
              frame False {
              }
              frame True {
                n2507 = local write "Rt 3"(FALSE ("Rt 3")) -> ()
              }
            }
            "Rt" <- TRUE ("Rt")
            "Rt 2" <- FALSE ("Rt")
          }
          frame True {
            n2508 = local read "Rt"() -> (w3004:bool)
            n2509 = local write "Rt 2"(TRUE ("Rt 2")) -> ()
            n2510 = case shown="True" w3004 {
              frame False {
              }
              frame True {
                n2511 = local write "Rt"(FALSE ("Rt")) -> ()
              }
            }
            "Rt 3" <- TRUE ("Rt 3")
          }
        }
        n2512 = case shown="\"Acquire\"" w2931 {
          tunnel: w2933 -> [_ w3033]
          frame Default {
            w3032 = 0.0 ("output")
            n2513 = local write "PID-out"(w3032) -> ()
            n2514 = local write "Frequency ( Hz )"(w3032) -> ()
            n2515 = local write "STROKE Initialize"(TRUE ("STROKE Initialize")) -> ()
          }
          frame "Acquire" {
            n2516 = stacked-sequence {
              frame #0 {
                n2517 = local read "Auto Start Test"() -> (w3035:bool)
                n2518 = case shown="True" w3035 {
                  tunnel: "RUN" -> [w3056 w3059]
                  tunnel: [w3056 w3058] -> w3036
                  frame False {
                  }
                  frame True {
                    n2519 = local read "Auto Start Temp"() -> (w3057:bool)
                    n2520 = Or(x=w3059, y=w3057) -> (x .or. y?=w3058:bool)
                  }
                }
                n2521 = local read "clk"() -> (w3055:dbl)
                n2522 = local read "Save"() -> (w3051:bool)
                n2523 = Equal?(x=w3055, y=0.0) -> (x = y?=w3052:bool)
                n2524 = And(x=w3052, y=w3051) -> (x .and. y?=w3053:bool)
                n2525 = Not(x="Engage") -> (.not. x?=w3042:bool)
                n2526 = case shown="False" w3036 {
                  tunnel: [0.0 w3083] -> w3038
                  frame False {
                    (unwired) TRUE ("Visible")
                    n2527 = local read "Auto Start Test"() -> (w3063:bool)
                    n2528 = local write "Start Time"(TRUE ("Start Time")) -> ()
                    n2529 = property on="Stroke 2" class="DigNum (strict)"("Visible"=FALSE) -> ()  [unwired: 2 in, 2 out]
                    n2530 = case shown="False" w3063 {
                      frame False {
                        n2531 = property on="Heater Button" class="Bool (strict)"("DisabledEnum"=T19."Enabled" ("Disabled")) -> ()  [unwired: 2 in, 2 out]
                        n2532 = property on="Humidity" class="Bool (strict)"("DisabledEnum"=T19."Enabled" ("Disabled")) -> ()  [unwired: 2 in, 2 out]
                      }
                      frame True {
                      }
                    }
                    n2533 = case shown="False" "TestCompFlg" {
                      frame False {
                        n2534 = local read "StartFlg"() -> (w3071:bool)
                        n2535 = case shown="True" w3071 {
                          frame False {
                          }
                          frame True {
                            n2536 = stacked-sequence {
                              frame #0 {
                                n2537 = local read "EVENT LOG"() -> (w3075:string)
                                n2538 = call "Event Log.vi"("Content"="Test was interrupted", "EVENT LOG"=w3075) -> ("EVENT LOG"=w3076:string)  [unwired: 8 in, 1 out]
                                n2539 = local write "EVENT LOG"(w3076) -> ()
                                n2540 = property on="RUN" class="Bool (strict)"("Visible"=TRUE) -> ()  [unwired: 2 in, 2 out]
                                n2541 = property on="Auto Start Test" class="Bool (strict)"("Visible"=TRUE) -> ()  [unwired: 2 in, 2 out]
                              }
                              frame #1 {
                                w3079 = FALSE ("StartFlg")
                                n2542 = property on="Heater Button" class="Bool (strict)"("Val(Sgnl)"=FALSE ("Value (Signaling)")) -> ()  [unwired: 2 in, 2 out]
                                n2543 = local write "Heater Button"(w3079) -> ()
                                n2544 = local write "StartFlg"(w3079) -> ()
                                n2545 = local write "Humidity"(w3079) -> ()
                                n2546 = local write "Humidity"(TRUE ("Humidity")) -> ()
                              }
                              frame #2 {
                                n2547 = local write "Due Write"("VC;0" ("Command")) -> ()
                              }
                              frame #3 {
                                n2548 = Wait (ms)(milliseconds to wait=u32 1500) -> ()  [unwired: 1 out]
                              }
                              frame #4 {
                                n2549 = local write "Due Write"("HE;0" ("Command")) -> ()
                              }
                            }
                          }
                        }
                      }
                      frame True {
                      }
                    }
                    n2550 = local write "String 14"("Test will autostart once parameters reach the set value." ("String 14")) -> ()
                  }
                  frame True {
                    (unwired) FALSE ("Visible")
                    n2551 = property on="Stroke 2" class="DigNum (strict)"("Visible"=TRUE) -> ()  [unwired: 2 in, 2 out]
                    n2552 = property on="STOP 2" class="Bool (strict)"("Disabled"=u8 2) -> ()  [unwired: 2 in, 2 out]
                    n2553 = local write "String 14"(" Running....." ("String 14")) -> ()
                    n2554 = property on="Heater Button" class="Bool (strict)"("DisabledEnum"=T19."Disabled and Grayed Out" ("Disabled")) -> ()  [unwired: 2 in, 2 out]
                    n2555 = property on="Humidity" class="Bool (strict)"("DisabledEnum"=T19."Disabled and Grayed Out" ("Disabled")) -> ()  [unwired: 2 in, 2 out]
                    n2556 = case shown="True" "Start Time" {
                      selector: "Start Time" -> [_ w3102]
                      frame False {
                      }
                      frame True {
                        n2557 = Not(x=w3102) -> (.not. x?=w3101:bool)
                        n2558 = local write "Start Time"(w3101) -> ()
                        n2559 = local read "EVENT LOG"() -> (w3103:string)
                        n2560 = call "Event Log.vi"("Content"="Test in progress", "EVENT LOG"=w3103) -> ("EVENT LOG"=w3105:string)  [unwired: 8 in, 1 out]
                        n2561 = local write "EVENT LOG"(w3105) -> ()
                      }
                    }
                    n2562 = disable-structure shown="Enabled" {
                      disable-tunnel: [w3094 w3100] -> w3083
                      frame Disabled {
                        n2563 = local read "Set Hz"() -> (w3097:dbl)
                        n2564 = call <vilib>:"Uniform White Noise Waveform.vi"() -> ("signal out"=w3096:waveform(dbl))  [unwired: 10 in, 1 out]
                        n2565 = Random Number (0-1)() -> (number: 0 to 1=w3093:dbl)
                        n2566 = Add(x=w3097, y=w3096) -> (x+y=w3095:waveform(dbl))
                        n2567 = Multiply(x=ext 0.01 ("y"), y=w3093) -> (x*y=w3091:ext)
                        n2568 = Multiply(x=w3095, y=w3091) -> (x*y=w3094:waveform(ext))
                      }
                      frame Enabled {
                        n2569 = call-poly <vilib>:"Random Number (Range).vi"("lower bound (0)"=49.89, "upper bound (100)"=50.8) -> ("number"=w3100:dbl)  [unwired: 9 in]
                      }
                    }
                    "StartFlg" <- TRUE ("StartFlg")
                  }
                }
                n2570 = case shown="True" w3053 {
                  frame False {
                  }
                  frame True {
                    n2571 = local write "clk"(10.0 ("clk")) -> ()
                    n2572 = Get Date/Time In Seconds() -> (seconds since 1Jan1904=w3108:timestamp)
                    n2573 = To Double Precision Float(number=w3108) -> (double precision float=w3106:dbl)
                    n2574 = local write "acq timer"(w3106) -> ()
                    n2575 = local write "act save time"(w3106) -> ()
                  }
                }
                n2576 = call "Elapsed Time"("Time Target (s)"="Countdown", "Reset"=w3042) -> ("Elapsed Time (s)"=w3047:dbl, "Time has Elapsed"=w3045:bool)  [unwired: 10 in, 6 out]
                "Countdown 2" <- w3047
                n2577 = Subtract(x=w3047, y=2.0) -> (x-y=w3050:dbl)
                n2578 = Less?(x=w3050, y="Countdown") -> (x < y?=w3048:bool)
                n2579 = And(x=w3048, y=w3045) -> (x .and. y?=w3044:bool)
                n2580 = case shown="True" w3044 {
                  frame False {
                  }
                  frame True {
                    (unwired) dbl[] [] ("History Data")
                    n2581 = local write "Engage"(FALSE ("Engage")) -> ()
                    n2582 = local write "RUN"(TRUE ("RUN")) -> ()
                    n2583 = local read "Humidity ( %RH )"() -> (→"Rh Before":dbl)
                  }
                }
                n2584 = local read "Test \nStatus"() -> (w3040:bool)
                n2585 = Select(t=w3038, s=w3040, f=0.0) -> (s? t:f=w3039:dbl)
                n2586 = local write "Frequency ( Hz )"(w3039) -> ()
              }
              frame #1 {
                w3131 = 1000000.0 ("x")
                # "HC;1/0\nST;VALUE"
                # "Elapsed time\ncof\nstroke\nAir temp\nTemp\nHumidity"
                # "acq timer\n\nact save time"
                # "convert to microseconds"
                n2587 = local read "COUNT"() -> (w3114:i32)
                n2588 = local read "Rate"() -> (w3127:dbl)
                n2589 = Divide(x=w3131, y=w3127) -> (x/y=w3132:dbl)
                n2590 = Greater Or Equal?(x=w3114, y=250) -> (x >= y?=w3113:bool)
                n2591 = Get Date/Time In Seconds() -> (seconds since 1Jan1904=w3134:timestamp)
                n2592 = case shown="True" w3113 {
                  frame False {
                    n2593 = local read "COUNT"() -> (w3135:i32)
                    n2594 = Increment(x=w3135) -> (x+1=w3136:i32)
                    n2595 = local write "COUNT"(w3136) -> ()
                  }
                  frame True {
                    n2596 = local write "COUNT"(0 ("COUNT")) -> ()
                  }
                }
                n2597 = local read "Samplingtime 2"() -> (w3112:dbl)
                n2598 = local read "act save time"() -> (w3129:dbl)
                n2599 = Divide(x=w3132, y=w3131) -> (x/y=w3130:dbl)
                n2600 = To Double Precision Float(number=w3134) -> (double precision float=w3123:dbl)
                n2601 = Add(x=w3129, y=w3112) -> (x+y=w3128:dbl)
                n2602 = local read "acq timer"() -> (w3133:dbl)
                n2603 = local read "COUNT"() -> (w3116:i32)
                n2604 = Greater Or Equal?(x=w3123, y=w3128) -> (x >= y?=w3111:bool)
                n2605 = Multiply(x=w3130, y=w3116) -> (x*y=w3122:dbl)
                n2606 = Subtract(x=w3123, y=w3133) -> (x-y=w3125:dbl)
                n2607 = local read "Save"() -> (w3126:bool)
                n2608 = Add(x=w3125, y=w3122) -> (x+y=w3109:dbl)
                "Elapsed time 3" <- w3109
                n2609 = And(x=w3111, y=w3126) -> (x .and. y?=w3124:bool)
                n2610 = Divide(x=w3109, y=60.0) -> (x/y=w3120:dbl)
                n2611 = local read "Test \nStatus"() -> (w3110:bool)
                n2612 = local read "clk"() -> (w3117:dbl)
                n2613 = Equal?(x=w3117, y=10.0) -> (x = y?=w3119:bool)
                n2614 = case shown="True" w3124 {
                  tunnel: w3123 -> [_ w3250]
                  tunnel: [FALSE ("Boolean 2") TRUE ("Boolean 2")] -> _
                  frame False {
                  }
                  frame True {
                    w3204 = ";" ("Substring")
                    # "Pid out/\nFreq response value"
                    n2615 = local write "act save time"(w3250) -> ()
                    n2616 = local read "FILE"() -> (w3198:string)
                    n2617 = call "file check.vi"("file name in"=w3198) -> ("error out"=w3201:errorcluster, "file name out"=w3196:string)  [unwired: 9 in]
                    n2618 = local read "LVDT STROKE"() -> (w3193:dbl)
                    n2619 = local read "Add up Stroke"() -> (w3191:dbl)
                    n2620 = call "FILE PATH CREATION.vi"("error in"=w3201, "FILE NAME :"=w3196) -> ("FILE OUT"=w3199:path)  [unwired: 8 in, 1 out]
                    n2621 = local read "STROKE Initialize"() -> (w3186:bool)
                    n2622 = Concatenate Strings(w3196, ".dgf" ("Substring")) -> (w3200:string)
                    n2623 = Subtract(x=w3193, y=w3191) -> (x-y=w3192:dbl)
                    n2624 = Absolute Value(x=w3192) -> (abs(x)=w3189:dbl)
                    n2625 = local read "FF 2"() -> (→"Frictional Force ( N )" →"Frictional Force ( N )":dbl)
                    n2626 = Build Path(base path=w3199, name or relative path=w3200) -> (appended path=w3195:path)
                    n2627 = flat-sequence {
                      tunnel: w3189 -> [w3255]
                      tunnel: [w3254] -> w3187
                      tunnel: w3186 -> [w3252]
                      tunnel: [w3257] -> w3188
                      tunnel: w3187 -> [w3257]
                      frame #0 {
                        n2628 = call <vilib>:"Mean PtByPt.vi"("x"=w3255, "sample length"="STROKE FILTER", "initialize"=w3252) -> ("mean"=w3254:dbl)  [unwired: 1 in, 1 out]
                      }
                      frame #1 {
                        "STROKE Initialize" <- FALSE ("STROKE Initialize")
                      }
                    }
                    n2629 = local read "COF 2"() -> (w3209:dbl)
                    "Coefficient of Friction" <- w3209
                    "COF 4" <- w3209
                    "Coefficient of Friction" <- w3209
                    n2630 = local read "TEMP"() -> (w3212:dbl)
                    "Temperature ( Deg C )" <- w3212
                    n2631 = local read "Humidity ( %RH )"() -> (w3211:dbl)
                    n2632 = local read "Frequency ( Hz )"() -> (w3218:dbl)
                    n2633 = local read "LVDT STROKE DISPLAY"() -> (w3190:dbl)
                    n2634 = local read "Elapsed time"() -> (w3243:dbl)
                    n2635 = local read "AIR TEMP"() -> (w3216:dbl)
                    n2636 = local read "PID-out"() -> (w3221:dbl)